vi "UHR-Fleezers Control (host) - 10.4.vi"() -> ()   [LabVIEW 2010] (continued)
  n62 = local read "Scan BD"() -> (w215:bool)
  n63 = And(x=w231, y=w232) -> (x .and. y?=w230:cluster{"Set 1":bool, "Set 2":bool})
  n64 = local write "Data points/scan (f/b)"(w200) -> ()
  n65 = Reciprocal(x=w167) -> (1/x=w168:dbl)
  n66 = local read "N Acq Sets (Traps + Fl.)"() -> (w159:i16)
  n67 = local write "N sets should be saved"(w196) -> ()
  n68 = Unbundle By Name(w230) -> ("Set 1"=w234:bool, "Set 2"=w233:bool)
  n69 = local read "Interlace"() -> (w96:bool)
  n70 = Select(t=w103, s=w96, f=w101) -> (s? t:f=w93:u32)
  n71 = local write "Update Count (MCL)"(w93) -> ()
  n72 = local write "Total Counts (ticks)"(w93) -> ()
  n73 = xnode "Invoke Method"("FPGA VI Reference In"=w220, "error in"=w219) -> ("FPGA VI Reference Out"=w112:T20, "error out"=w133:errorcluster)
  n74 = local write "Ave. Period (s)"(w168) -> ()
  n75 = property on="2D or 1D Scan" class="Bool (strict)"("Val(Sgnl)"=w114) -> ()  [unwired: 2 in, 2 out]
  n76 = xnode "Read/Write Control"("FPGA VI Reference In"=w111, "error in"=w133, "ai count"="AI Count (ticks)", "Interlace ON/OFF"=w96, "Number Interlace Cycles"=w95, "AI1 Sets to FIFO"=w235, "FB On/Off Set 1"=w234, "FB On/Off Set 2"=w233, "Interlace Off Parameters"=w94, "FB Setpoint Set 1"=w225, "FB Setpoint Set 2"=w224, "FB Gains Set 1"=w222, "FB Gains Set 2"=w221, "FB output range 1"=w113, "FB output range 2"=w113, "Cycles per step"=w203, "Scan BD"=w215, "Number of scans"=w199, "Scan steps"=w204, "Scan freq.  increment"=w205, "AO1"=w187, "AO2"=w186, "Scan freq.  increment (MCL)"=w180, "Scan steps (MCL)"=w179, "Cycles per step (MCL)"=w178, "Number of scans (MCL)"=w177, "MCL count"=w93, "Cont. Scan (MCL)"=w176, "MCL Scan Axis"=w170, "1D or 2D Scan?"=w114, "N of AI1 Int Acq Sets"=w159, "Freq or Amp switch first"="Freq or Amp switch first", "Freq switch delay"="Freq switch delay", "Amp switch delay"="Amp switch delay", "Swap F1 and F2"="Swap F1 and F2", "APD Acq Rate Count"=w119, "APD to FIFO"=FALSE, "APD Gate Operating Mode"="APD Gate", "APD Gate ON Count"="APD Gate ON Count", "APD Gate OFF Count"="APD Gate OFF Count", "Invert APD Gate"="Invert APD Gate", "DIO count 1 (ticks)"="DIO count 1 (ticks)", "DIO count 2 (ticks)"="DIO count 2 (ticks)", "DIO count 3 (ticks)"="DIO count 3 (ticks)", "APD 1 AO scale factor"="APD 1 AO Mult.", "APD 2 AO scale factor"="APD 2 AO Mult.") -> ("FPGA VI Reference Out"=w88:T20, "error out"=w90:errorcluster)  [unwired: 1 in]
  n77 = local read "Green Laser ON/Interlacing"() -> (w91:bool)
  n78 = local read "Green laser mode"() -> (w92:enum32{"Laser ON", "Laser OFF", "Interlace"})
  n79 = local read "GI Frequency, OFF count"() -> (w84:u32)
  n80 = local read "GI Frequency, ON count"() -> (w83:u32)
  n81 = Multiply(x="Current When FB OFF (%)", y=655.35) -> (x*y=w74:dbl)
  n82 = local read "Green FB Count"() -> (w82:u32)
  n83 = Multiply(x="Green FB Setpoint (mV)", y=3.2767) -> (x*y=w71:dbl)
  n84 = To Unsigned Word Integer(number=w74) -> (unsigned 16bit integer=w72:u16)
  n85 = local read "Invert GI"() -> (w86:bool)
  n86 = To Word Integer(number=w71) -> (16bit integer=w69:i16)
  n87 = case shown="False" w91 {
    tunnel: w92 -> [_ w261]
    tunnel: [enum32{"Laser ON", "Laser OFF", "Interlace"}."Laser OFF" ("Green laser mode") w261] -> w85
    frame False {
    }
    frame True {
    }
  }
  n88 = local read "Trap Pos. AI1 X Pre-scale"() -> (w31:u16)
  n89 = local read "Trap Pos FB Monitor\nT1 or T2"() -> (w38:bool)
  n90 = local read "Trap Pos FB Int Count"() -> (w26:u16)
  n91 = local read "Trap Pos FB Negate Action"() -> (w37:bool)
  n92 = local read "Trap Pos. FB Offset Factor"() -> (w36:i64)
  n93 = local read "Trap Pos. FB Mult Factor"() -> (w35:i64)
  n94 = local read "Trap Pos. FB Gains"() -> (w33:T12)
  n95 = local read "Trap Pos. FB Range"() -> (w34:T13)
  n96 = xnode "Read/Write Control"("FPGA VI Reference In"=w88, "error in"=w90, "Green interlace ON count 2"=w83, "Green interlace OFF count 2"=w84, "Invert GI 2"=w86, "Operating Mode 2"=w85, "Green FB Gains"="Green FB Gains", "Green FB Setpoint"=w69, "Green FB On/Off"="Green FB On/Off", "Current Out"=w72, "Green int current ON count adj"="Green int current ON count adj", "Green FB Count"=w82, "Operating Mode"=w85, "Green interlace OFF count"=w84, "Green interlace ON count"=w83, "Invert GI"=w86, "Trap Pos FB Monitor T1 or T2"=w38, "Trap Pos FB Negate Action"=w37, "Trap Pos. FB Offset Factor"=w36, "Trap Pos. FB Mult Factor"=w35, "Trap Pos. FB Range"=w34, "Trap Pos. FB Gains"=w33, "Force feedback"=FALSE, "AI1 X Scale"=w31, "Trap Pos to FIFO"=TRUE, "Trap Pos FB Int Count"=w26) -> ("FPGA VI Reference Out"=w87:T20, "error out"=w89:errorcluster)
  n97 = xnode "Invoke Method"("FPGA VI Reference In"=w87, "error in"=w89, "Depth"="Trap AI FIFO Depth") -> ("FPGA VI Reference Out"=w41:T20, "error out"=w40:errorcluster)
  n98 = xnode "Invoke Method"("FPGA VI Reference In"=w41, "error in"=w40, "Depth"="Trap Position FIFO Depth") -> ("FPGA VI Reference Out"=w28:T20, "error out"=w27:errorcluster)
  n99 = flat-sequence {
    tunnel: w112 -> [w266]
    tunnel: [w266] -> w111
    tunnel: [w265] -> w110
    tunnel: [w264] -> w109
    tunnel: [w262] -> w107
    tunnel: [w263] -> w108
    frame #0 {
      w263 = T17 {"Minimum"=0.0, "Maximum"=40.0, "Increment"=1.0} ("Min Max Inc")
      w262 = T17 {"Minimum"=0.0, "Maximum"=50.0, "Increment"=1.0} ("Data Entry Limits")
      w265 = T17 {"Minimum"=60.0, "Maximum"=90.0, "Increment"=1.0} ("Min Max Inc")
      w264 = T17 {"Minimum"=0.0, "Maximum"=50.0, "Increment"=1.0} ("Data Entry Limits")
      n100 = property on="BD 2 Frequency 1 (MHz)" class="DigNum (strict)"("Data Range"=w263) -> ()  [unwired: 2 in, 2 out]
      n101 = property on="BD 2 Frequency 3 (MHz)" class="DigNum (strict)"("Data Range"=w263) -> ()  [unwired: 2 in, 2 out]
      n102 = property on="BD 2 Frequency 2 (MHz)" class="DigNum (strict)"("Data Range"=w263) -> ()  [unwired: 2 in, 2 out]
      n103 = property on="BD 1 Frequency 1 (MHz)" class="DigNum (strict)"("Data Range"=w265) -> ()  [unwired: 2 in, 2 out]
      n104 = property on="BD 1 Frequency 2 (MHz)" class="DigNum (strict)"("Data Range"=w265) -> ()  [unwired: 2 in, 2 out]
      n105 = property on="BD 1 Frequency 3 (MHz)" class="DigNum (strict)"("Data Range"=w265) -> ()  [unwired: 2 in, 2 out]
      n106 = property on="BD 2 Amplitude 1 (%)" class="DigNum (strict)"("Data Range"=w262) -> ()  [unwired: 2 in, 2 out]
      n107 = property on="BD 2 Amplitude 2 (%)" class="DigNum (strict)"("Data Range"=w262) -> ()  [unwired: 2 in, 2 out]
      n108 = property on="BD 2 Amplitude 3 (%)" class="DigNum (strict)"("Data Range"=w262) -> ()  [unwired: 2 in, 2 out]
      n109 = property on="BD 1 Amplitude 3 (%)" class="DigNum (strict)"("Data Range"=w264) -> ()  [unwired: 2 in, 2 out]
      n110 = property on="BD 1 Amplitude 2 (%)" class="DigNum (strict)"("Data Range"=w264) -> ()  [unwired: 2 in, 2 out]
      n111 = property on="BD 1 Amplitude 1 (%)" class="DigNum (strict)"("Data Range"=w264) -> ()  [unwired: 2 in, 2 out]
      "X RF Frequency Limits (MHz)" <- w265
      "X RF Amplitude Limits (%)" <- w264
      "Y RF Amplitude Limits (%)" <- w262
      "Y RF Frequency Limits (MHz)" <- w263
    }
  }
  n112 = xnode "Invoke Method"("FPGA VI Reference In"=w28, "error in"=w27) -> ("FPGA VI Reference Out"=w132:T20, "error out"=w131:errorcluster)  [unwired: 1 out]
  n113 = flat-sequence "Initial FPGA Loop Relative Phase Adjustment" {
    tunnel: "Initial Phase Adjustment (AI1)" -> [w277]
    tunnel: "Initial Phase Adjustment (GI)" -> [w276]
    tunnel: w132 -> [w275]
    tunnel: w131 -> [w274]
    tunnel: "Initial Phase Adj. (MCL)" -> [w273]
    tunnel: [w278] -> w141
    tunnel: [w272] -> w137
    tunnel: "Initial Phase Adjustment (APD Acq)" -> [w271]
    tunnel: "Initial Phase Adjustment (APD 1 Gate)" -> [w270]
    tunnel: "Initial Phase Adjustment (Green FB)" -> [w269]
    tunnel: "Initial Phase Adjustment (GI) 2" -> [w268]
    tunnel: "Initial Phase Adjustment (APD 2 Gate)" -> [w267]
    tunnel: w141 -> [w457]
    tunnel: [w458] -> w138
    tunnel: w137 -> [w458]
    tunnel: [w457] -> w136
    tunnel: w138 -> [w461]
    tunnel: w136 -> [w460]
    tunnel: [w463] -> w135
    tunnel: [w462] -> w134
    tunnel: [w650] -> w139
    tunnel: [w651] -> w140
    tunnel: w135 -> [w651]
    tunnel: w134 -> [w650]
    frame #0 {
      n114 = xnode "Read/Write Control"("FPGA VI Reference In"=w275, "error in"=w274, "Phase count adjustment"=w277, "Phase count adjustment (GI)"=w276, "Phase count adjustment (MCL)"=w273, "Phase Count Adjustment (APD Acq)"=w271, "Phase count adjustment (APD 1 Gate)"=w270, "Phase count adjustment (APD 2 Gate)"=w267, "Phase count adjustment (Green FB)"=w269, "Phase count adjustment (GI) 2"=w268) -> ("FPGA VI Reference Out"=w272:T20, "error out"=w278:errorcluster)
    }
    frame #1 {
      n115 = Wait (ms)(milliseconds to wait=u32 100) -> ()  [unwired: 1 out]
    }
    frame #2 {
      w459 = TRUE
      n116 = xnode "Read/Write Control"("FPGA VI Reference In"=w461, "error in"=w460, "+ phase"=w459, "+ phase (GI)"=w459, "+ phase (MCL)"=w459, "+ phase (APD Acq)"=w459, "+ phase (APD 1 Gate)"=w459, "+ phase (APD 2 Gate)"=w459, "+ phase (Green FB)"=w459, "+ phase (GI) 2"=w459) -> ("FPGA VI Reference Out"=w462:T20, "error out"=w463:errorcluster)
    }
    frame #3 {
      n117 = Wait (ms)(milliseconds to wait=u32 100) -> ()  [unwired: 1 out]
    }
  }
  n118 = local read "Phase adj. (Green FB)"() -> (w105:i16)
  n119 = local read "Phase adj. (GI) 2"() -> (w75:i16)
  n120 = local read "Phase adjust (MCL)"() -> (w171:i16)
  n121 = local read "Phase adj. (AI1)"() -> (w173:i16)
  n122 = local read "Phase adj. (GI)"() -> (w172:i16)
  n123 = xnode "Read/Write Control"("FPGA VI Reference In"=w139, "error in"=w140, "Phase count adjustment"=w173, "Phase count adjustment (GI)"=w172, "Phase count adjustment (MCL)"=w171, "Phase Count Adjustment (APD Acq)"="Phase Adj. (APD Acq)", "Phase count adjustment (APD 1 Gate)"="Phase Adj. (APD 1 Gate)", "Phase count adjustment (APD 2 Gate)"="Phase Adj. (APD 2 Gate)", "Phase count adjustment (Green FB)"=w105, "Phase count adjustment (GI) 2"=w75) -> ("FPGA VI Reference Out"=w61:T20, "error out"=w148:errorcluster)
  n124 = call "Initialize RF boards - interlace 3.vi"("error in"=w148, "FPGA VI Reference In"=w61) -> ("error out"=w146:errorcluster, "FPGA VI Reference Out"=w147:T20)
  n125 = call "set RF board frequency - interlace.vi"("Board 2 Frequency Limits"=w108, "Board 1 Frequency Limits"=w110, "error in"=w146, "FPGA VI Reference In"=w147, "Board 2 Frequency 3 (MHz)"="BD 2 Frequency 3 (MHz)", "Board 1 Frequency 3 (MHz)"="BD 1 Frequency 3 (MHz)", "Board 2 Frequency 2 (MHz)"="BD 2 Frequency 2 (MHz)", "Board 2 Frequency 1 (MHz)"="BD 2 Frequency 1 (MHz)", "Board 1 Frequency 2 (MHz)"="BD 1 Frequency 2 (MHz)", "Board 1 Frequency 1  (MHz)"="BD 1 Frequency 1 (MHz)") -> ("error out"=w250:errorcluster, "FPGA VI Reference Out"=w251:T20)
  n126 = call "set RF board amplitude - interlace.vi"("Board 2 Amplitude Limits"=w107, "Board 1 Amplitude Limits"=w109, "error in"=w250, "FPGA VI Reference In"=w251, "Board 2 Amplitude 3 (%)"="BD 2 Amplitude 3 (%)", "Board 1 Amplitude 3 (%)"="BD 1 Amplitude 3 (%)", "Board 2 Amplitude 2 (%)"="BD 2 Amplitude 2 (%)", "Board 2 Amplitude 1 (%)"="BD 2 Amplitude 1 (%)", "Board 1 Amplitude 2 (%)"="BD 1 Amplitude 2 (%)", "Board 1 Amplitude 1 (%)"="BD 1 Amplitude 1 (%)") -> ("error out"=w238:errorcluster, "FPGA VI Reference Out"=w239:T20)
  n127 = flat-sequence {
    tunnel: w239 -> [w660]
    tunnel: w238 -> [w659]
    tunnel: [w658] -> w243
    tunnel: [w657] -> w242
    tunnel: [w702] -> w241
    tunnel: w243 -> [w702]
    tunnel: [w701] -> w240
    tunnel: w242 -> [w701]
    tunnel: w241 -> [w711]
    tunnel: w240 -> [w710]
    tunnel: [w709] -> w20
    tunnel: [w708] -> w19
    tunnel: [w766] -> w21
    tunnel: [w776] -> w18
    tunnel: w20 -> [w776]
    tunnel: w19 -> [w771]
    frame #0 {
      n128 = local read "Trap 1 (ON/OFF)"() -> (w652:bool)
      n129 = xnode "Read/Write Control"("FPGA VI Reference In"=w660, "error in"=w659, "Direct RF Box  Communication"=FALSE) -> ("FPGA VI Reference Out"=w658:T20, "error out"=w657:errorcluster)
      n130 = local write "Saving..."(FALSE ("Saving Data")) -> ()
      n131 = local write "Stop All"(FALSE ("Stop All")) -> ()
      n132 = local write "Index"(1.0 ("Index")) -> ()
      n133 = property on="Trap 1 ON" class="Bool (strict)"("Value"=w652) -> ()  [unwired: 2 in, 2 out]
      "Manipulating Trap" <- FALSE ("Manipulating Trap")
    }
    frame #1 {
      n134 = local read "Trap 2 (ON/OFF)"() -> (w700:bool)
      n135 = Wait (ms)(milliseconds to wait=u32 10) -> ()  [unwired: 1 out]
      n136 = property on="Trap 2 ON" class="Bool (strict)"("Val(Sgnl)"=w700) -> ()  [unwired: 2 in, 2 out]
    }
    frame #2 {
      n137 = local read "Scan Range (nm)"() -> (w704:dbl)
      n138 = xnode "Read/Write Control"("FPGA VI Reference In"=w711, "error in"=w710, "FPGA Controls  RF Box"=TRUE ("Direct RF Box  Communication")) -> ("FPGA VI Reference Out"=w709:T20, "error out"=w708:errorcluster)
      n139 = call "Update messages.vi"("Message to add"="UHR-Fleezers ready.", "Old message string"="") -> ("New message string"=w707:string)
      n140 = local write "Messages"(w707) -> ()
      n141 = property on="Scan Range (nm)" class="DigNum (strict)"("Val(Sgnl)"=w704) -> ()  [unwired: 2 in, 2 out]
    }
    frame #3 {
      w754 = T23."ASCII" ("Command")
      # "disable hysteresis\ncompensation for\nfaster performance"
      # "increase jerk\nfor faster \nresponse"
      # "disable backlash\ncompensation for\nfaster response \ntimes. necessary\nfor mouse control\nof stage"
      n142 = call "CONEX_FUNCTIONAL_GLOBAL.vi"("error in"=w771, "Command"=T23."INIT") -> ("error out"=w768:errorcluster)  [unwired: 7 in, 2 out]
      n143 = call "CONEX_FUNCTIONAL_GLOBAL.vi"("error in"=w768, "Position"=dbl[] [10.0, 12.0, 6.025], "Command"=T23."SET ULIM") -> ("error out"=w772:errorcluster)  [unwired: 6 in, 2 out]
      n144 = call "CONEX_FUNCTIONAL_GLOBAL.vi"("error in"=w772, "Position"=dbl[] [4.0, 0.0, 5.8], "Command"=T23."SET LLIM") -> ("error out"=w764:errorcluster)  [unwired: 6 in, 2 out]
      n145 = Concatenate Strings("1BA0", "\r\n") -> (w761:string)
      n146 = call "CONEX_FUNCTIONAL_GLOBAL.vi"("error in"=w764, "ASCII command"=w761, "Command"=w754) -> ("error out"=w760:errorcluster)  [unwired: 6 in, 2 out]
      n147 = Concatenate Strings("1JR0.001", "\r\n") -> (w757:string)
      n148 = call "CONEX_FUNCTIONAL_GLOBAL.vi"("error in"=w760, "ASCII command"=w757, "Command"=w754) -> ("error out"=w756:errorcluster)  [unwired: 6 in, 2 out]
      n149 = Concatenate Strings("1BH0", "\r\n") -> (w751:string)
      n150 = call "CONEX_FUNCTIONAL_GLOBAL.vi"("error in"=w756, "ASCII command"=w751, "Command"=w754) -> ("error out"=w755:errorcluster)  [unwired: 6 in, 2 out]
      n151 = call "CONEX_FUNCTIONAL_GLOBAL.vi"("error in"=w755, "Command"=T23."GET POS") -> ("error out"=w766:errorcluster, "Current Position"=w765:dbl[])  [unwired: 7 in, 1 out]
      n152 = local write "Current Position"(w765) -> ()
    }
  }
  n153 = Subtract(x="BD 1 Frequency 1 (MHz)", y="BD 1 Frequency 2 (MHz)") -> (x-y=w158:dbl)
  n154 = Subtract(x="BD 2 Frequency 1 (MHz)", y="BD 2 Frequency 2 (MHz)") -> (x-y=w157:dbl)
  n155 = Square(x=w157) -> (x^2=w155:dbl)
  n156 = Square(x=w158) -> (x^2=w156:dbl)
  n157 = Add(x=w156, y=w155) -> (x+y=w154:dbl)
  n158 = Square Root(x=w154) -> (sqrt(x)=w153:dbl)
  n159 = local write "Trap Delta (MHz)"(w153) -> ()
  n160 = call "IMAQ Create"("Image Name"="APD 1 Image", "Image Type"=w52) -> ("New Image"=w51:T2)  [unwired: 3 in, 1 out]
  n161 = call "IMAQ Create"("Image Name"="APD 2 Image", "Image Type"=w52) -> ("New Image"=w50:T2)  [unwired: 3 in, 1 out]
  n162 = call "IMAQ Create"("Image Name"="Det. X Image", "Image Type"=w52) -> ("New Image"=w49:T2)  [unwired: 3 in, 1 out]
  n163 = call "IMAQ Create"("Image Name"="Det. Y Image", "Image Type"=w52) -> ("New Image"=w48:T2)  [unwired: 3 in, 1 out]
  n164 = call-poly "VISA Configure Serial Port"("VISA resource name"="Harvard Syringe Pump Serial Port", "baud rate (9600)"=u32 115200, "stop bits (10: 1 bit)"=w45) -> ("VISA resource name out"=w42:refnum<visa-resource-name>, "error out"=w43:errorcluster)  [unwired: 4 in, 7 out]
  n165 = Bundle("New Image"=w51, "New Image"=w50, "New Image"=w49, "New Image"=w48) -> (w47:T24)  [unwired: 1 in]
  n166 = Tick Count (ms)() -> (millisecond timer value=w22:u32)
  n167 = call <vilib>:"IMAQ Init.vi"("Interface Name"="img0") -> ("error out"=w13:errorcluster, "IMAQ Session Out"=w15:refnum<k11>)  [unwired: 9 in]
  n168 = call <vilib>:"IMAQ Grab Setup.vi"("error in (no error)"=w13, "IMAQ Session In"=w15) -> ("error out"=w9:errorcluster, "IMAQ Session Out"=w10:refnum<k11>)  [unwired: 8 in]
  n169 = call "IMAQ Create"("Image Name"="untitled", "Image Type"=w11) -> ("New Image"=w8:T2)  [unwired: 3 in, 1 out]
  n170 = call <vilib>:"Initialize Mouse.vi"() -> ("device ID"=w2:refnum<k1>)  [unwired: 10 in, 1 out]
  n171 = while {
    tunnel: w18 -> [_]
    tunnel: w2 -> [w780]
    tunnel: [w779] -> w1
    stop <- w778 stop-if-true
    n172 = event shown="[2] \"Use mouse to move stage\n(press any key to quit)\": Value Change" {
      selector: _ -> [_ _ _]
      dyn-events: _ -> [_ _ _]
      timeout: 1 -> [_ _ _]
      tunnel: w780 -> [w785 w786 w796]
      tunnel: [w785 w786 w792] -> w779
      tunnel: [_ w787 _] -> w778
      event Timeout {
        n173 = event-data() -> ()  [unwired: 1 in, 2 out]
        n174 = call "CONEX_FUNCTIONAL_GLOBAL.vi"("Axis"=enum16{"X", "Y", "Z", "XY", "XZ", "YZ", "XYZ"}."XYZ", "Command"=T23."GET POS") -> ("Current Position"=w782:dbl[])  [unwired: 7 in, 2 out]
        n175 = Array To Cluster(array=w782) -> (cluster=→"Waveform Chart":T5)
        n176 = local write "Current Position"(w782) -> ()
      }
      event "Stop All": Value Change {
        n177 = event-data() -> ()  [unwired: 1 in, 5 out]
        n178 = local read "Stop All"() -> (w787:bool)
      }
      event "Use mouse to move stage\n(press any key to quit)": Value Change {
        n179 = event-data() -> ()  [unwired: 1 in, 1 out]
        n180 = local write "Stage Moving"(TRUE ("Stage Moving")) -> ()
        n181 = call-poly <vilib>:"Acquire Input Data.vi"("device ID"=w796) -> ("device ID"=w793:refnum<k1>)  [unwired: 15 in, 3 out]
        n182 = node-c288() -> (w795:T25)  [unwired: 4 in]
        n183 = timed-loop {
          timing: w795 -> [_]
          timing-out: [_] -> w794
          tunnel: w793 -> [w826]
          tunnel: [w825] -> w792
          tunnel: [w800] -> w789
          stop <- w809 stop-if-true
          (unwired) 10
          # "put cursor somewhere\nwhere mouse clicks and \nmouse wheel moves won't\nbe heard by the window"
          # "SetCursorPos"
          n184 = node-c288() -> ()  [unwired: 1 in, 1 out]
          n185 = call-poly <vilib>:"Acquire Input Data.vi"("device ID"=w826, "key mode"=enum16{"RELATIVE", "ABSOLUTE"}."RELATIVE") -> ("device ID"=w825:refnum<k1>, "axis info"=w823:T28, "button info"=w813:T29)  [unwired: 14 in, 1 out]
          n186 = Cluster To Array(cluster=w823) -> (array=w821:i32[])
          n187 = Unbundle By Name(w813) -> ("button 1"=w812:bool, "button 2"=w811:bool, "button 3"=w810:bool)
          n188 = Compound Arithmetic op=MULTIPLY(invert 10000.0 ("value"), "mouse sensitivity", w821) -> (w819:dbl[])
          n189 = call "subVI_explode3array.vi"("Array"=w819) -> ("x"=w804:dbl, "y"=w803:dbl, "z"=w818:dbl)  [unwired: 12 in]
          n190 = case shown="False" "invert y?" {
            tunnel: w803 -> [w827 w829]
            tunnel: [w827 w828] -> w802
            frame False {
            }
            frame True {
              n191 = Negate(x=w829) -> (-x=w828:dbl)
            }
          }
          n192 = case shown="False" "invert x?" {
            tunnel: w804 -> [w830 w832]
            tunnel: [w830 w831] -> w801
            frame False {
            }
            frame True {
              n193 = Negate(x=w832) -> (-x=w831:dbl)
            }
          }
          n194 = Compound Arithmetic op=OR(w812, w811, w810) -> (w809:bool)
          n195 = Divide(x=w818, y=50.0) -> (x/y=w816:dbl)
          n196 = Build Array(w801, w802, w816) -> (w807:dbl[])
          n197 = Not(x=w809) -> (.not. x?=w808:bool)
          n198 = call "CONEX_FUNCTIONAL_GLOBAL.vi"("Axis"=enum16{"X", "Y", "Z", "XY", "XZ", "YZ", "XYZ"}."XYZ", "Position"=w807, "Command"=T23."REL MOVE") -> ("error out"=w800:errorcluster)  [unwired: 6 in, 2 out]
          n199 = local write "Stage Moving"(w808) -> ()
          n200 = dll-call lib="User32.dll" fn="SetCursorPos"(700, 45) -> ()  [unwired: 5 in, 3 out]
          n201 = node-c288() -> ()  [unwired: 1 in, 1 out]
        }
        n202 = node-c288(w794) -> ()  [unwired: 1 out]
        n203 = call "CONEX_FUNCTIONAL_GLOBAL.vi"("Axis"=enum16{"X", "Y", "Z", "XY", "XZ", "YZ", "XYZ"}."XYZ", "error in"=w789, "Command"=T23."GET POS") -> ("Current Position"=w788:dbl[])  [unwired: 6 in, 2 out]
        n204 = local write "Current Position"(w788) -> ()
      }
    }
  }
  n205 = node-c288() -> (w17:T25)  [unwired: 4 in]
  n206 = timed-loop "acquire video and stage position" {
    timing: w17 -> [_]
    timing-out: [_] -> w16
    tunnel: w10 -> [w845]
    tunnel: w9 -> [w844]
    tunnel: w8 -> [w843]
    tunnel: [w842] -> w5
    tunnel: [w837] -> w4
    tunnel: [w838] -> w3
    tunnel: w18 -> [_]
    stop <- w839 stop-if-true
    n207 = node-c288() -> ()  [unwired: 1 in, 1 out]
    n208 = call <vilib>:"IMAQ Grab Acquire.vi"("error in (no error)"=w844, "Image In"=w843, "IMAQ Session In"=w845) -> ("error out"=w838:errorcluster, "Image Out"=w837:T2, "IMAQ Session Out"=w842:refnum<k11>)  [unwired: 5 in, 1 out]
    "Primary Video Display" <- w837
    n209 = local read "Stop All"() -> (w840:bool)
    n210 = Unbundle By Name(w838) -> ("status"=w841:bool)
    n211 = Or(x=w841, y=w840) -> (x .or. y?=w839:bool)
    n212 = node-c288() -> ()  [unwired: 1 in, 1 out]
  }
  n213 = node-c288(i64 1 ("Period"), 1 ("Processor")) -> (w162:T25)  [unwired: 2 out]
  n214 = node-c288(2 ("Processor")) -> (w65:T25)  [unwired: 3 out]
  n215 = node-c288() -> (w57:T25)  [unwired: 4 in]
  n216 = node-c288() -> (w67:T25)  [unwired: 4 out]
  n217 = timed-loop "Acquire Data" {
    tunnel: w18 -> [w1112]
    tunnel: w21 -> [w1111]
    tunnel: [w1142] -> w258
    tunnel: [w1136] -> w256
    timing: w162 -> [_]
    timing-out: [_] -> w161
    tunnel: w47 -> [w940]
    shift-right: [w856] -> _
    shift-left: w22 -> [w858]
    stop <- "Stop All" stop-if-true
    (unwired) u32 0 ("Number of Elements")
    w927 = "NI_ChannelName" ("name")
    # "originally this was Trap AI FIFO Depth -\nTrap AI Elements/DMA read. The subtraction\nof zero is a kluge to make it work."
    n218 = node-c288() -> ()  [unwired: 2 out]
    n219 = Tick Count (ms)() -> (millisecond timer value=w856:u32)
    n220 = Tick Count (ms)() -> (millisecond timer value=w854:u32)
    n221 = First Call?() -> (First Call?: T/F=w893:bool)
    n222 = Subtract(x=w856, y=w858) -> (x-y=→"x-y":u32)
    n223 = Or(x="Reset", y=w893) -> (x .or. y?=w894:bool)
    n224 = flat-sequence {
      tunnel: w1112 -> [w1161]
      tunnel: w1111 -> [w1160]
      tunnel: w894 -> [w1157]
      tunnel: w854 -> [w1156]
      tunnel: [w1159] -> w851
      tunnel: [w1158] -> w850
      tunnel: [w1155] -> w849
      tunnel: [w1234] -> w853
      tunnel: [w1235] -> w1106
      tunnel: [w1236] -> w1107
      tunnel: w851 -> [w1236]
      tunnel: w850 -> [w1235]
      tunnel: w849 -> [w1234]
      tunnel: [w1233] -> w848
      frame #0 {
        n225 = case "Reset data stream" shown="True" w1157 {
          tunnel: w1161 -> [w1164 w1173]
          tunnel: w1160 -> [w1163 w1172]
          tunnel: [w1164 w1167] -> w1159
          tunnel: [w1163 w1166] -> w1158
          tunnel: w1156 -> [w1162 w1165]
          tunnel: [w1162 w1165] -> w1155
          frame False {
          }
          frame True {
            w1170 = TRUE ("AI to FIFO")
            n226 = local write "Overflow (data lost)"(FALSE ("Overflow (data lost)")) -> ()
            n227 = call "reset FPGA DMA.vi"("error in"=w1172, "FPGA VI Reference In"=w1173) -> ("error out"=w1168:errorcluster, "FPGA VI Reference Out"=w1169:T20)
            n228 = xnode "Read/Write Control"("FPGA VI Reference In"=w1169, "error in"=w1168, "AI to FIFO"=w1170, "APD to FIFO"=w1170) -> ("FPGA VI Reference Out"=w1167:T20, "error out"=w1166:errorcluster)
          }
        }
      }
      frame #1 {
        n229 = Tick Count (ms)() -> (millisecond timer value=w1233:u32)
      }
    }
    n230 = Or(x="Start AOD Scan", y="Trap Raster Scan") -> (x .or. y?=w1057:bool)
    n231 = case "Start AOM raster scan" shown="False" w1057 {
      tunnel: w1107 -> [w2785 w2795]
      tunnel: w1106 -> [w2784 w2794]
      tunnel: [w2785 w2788] -> w1105
      tunnel: [w2784 w2787] -> w1104
      frame False {
      }
      frame True {
        n232 = case shown="True" "Restart DMA? (AOD)" {
          tunnel: [w3206 w3208] -> w2789
          tunnel: [w3205 w3207] -> w2790
          tunnel: w2795 -> [w3206 w3210]
          tunnel: w2794 -> [w3205 w3209]
          frame False {
          }
          frame True {
            n233 = local write "Overflow (data lost)"(FALSE ("Overflow (data lost)")) -> ()
            n234 = call "reset FPGA DMA.vi"("error in"=w3209, "FPGA VI Reference In"=w3210) -> ("error out"=w3207:errorcluster, "FPGA VI Reference Out"=w3208:T20)
          }
        }
        n235 = local write "Trap Raster Scan"(FALSE ("Trap Raster Scan")) -> ()
        n236 = case shown="True" "Move MCL Also?" {
          tunnel: w2790 -> [w2798 w2907]
          tunnel: w2789 -> [w2799 w2908]
          tunnel: [w2797 w2911] -> w2788
          tunnel: [w2796 w2910] -> w2787
          frame False {
            w2800 = TRUE ("AI to FIFO")
            n237 = xnode "Read/Write Control"("FPGA VI Reference In"=w2799, "error in"=w2798, "AI to FIFO"=w2800, "APD to FIFO"=w2800, "Start scan"=w2800) -> ("FPGA VI Reference Out"=w2797:T20, "error out"=w2796:errorcluster)
          }
          frame True {
            w2904 = FALSE ("1D or 2D Scan?")
            w2909 = TRUE ("AI to FIFO")
            # "Count for MCL loop"
            # "N total cycles"
            # "N steps"
            # "V_int"
            n238 = local read "Scan Range (nm)"() -> (w2886:dbl)
            n239 = local read "Number of F/B Scans (AOD)"() -> (w2903:u16)
            n240 = Sign(1:w2886) -> (0:w2885:dbl)
            n241 = Compound Arithmetic op=MULTIPLY(w2886, "MCL Step Position Ratio", "MCL/AOM Scale Tweak") -> (w2890:dbl)
            n242 = Negate(x=w2885) -> (-x=w2882:dbl)
            n243 = Multiply(x=w2882, y="MCL Step Increment (V_int)") -> (x*y=w2884:dbl)
            n244 = Divide(x=w2890, y="MCL X Cal (nm/V)") -> (x/y=w2896:dbl)
            n245 = Multiply(x=32767.0 ("y"), y=w2896) -> (x*y=w2902:dbl)
            n246 = local read "Total Counts (ticks)"() -> (w2887:u32)
            n247 = local read "Cycles/step (AOD)"() -> (w2898:u64)
            n248 = local read "Scan steps (AOD)"() -> (w2899:u64)
            n249 = Divide(x=w2902, y=10.0) -> (x/y=w2895:dbl)
            n250 = Divide(x=w2895, y="MCL Step Increment (V_int)") -> (x/y=w2893:dbl)